vi "FRC ADIS16460 Example.vi"() -> ()   [LabVIEW 2015]
doc: "SimpleGyro Example\n\nThis example shows how to use a SimpleGyro sensor connected to the SPI port on the RoboRIO.\n\nThis example expects a USB cable connected from your development PC to the Type B USB Jack (next to the power input) on the roboRIO."
uses:
  <vilib>/Rock Robotics/SystemInterfaces/spilib/spi_bus.ctl
  ADI MXP IMU/FRC ADIS16460.lvlib
panel:
  out "IMU Data":T1
  out "IMU AHRS":cluster{"Pitch":dbl, "Roll":dbl}
  out "Sensor Ready?":bool
  out "IMU Angle Delta":cluster{"X":dbl, "Y":dbl, "Z":dbl}
  in  "Reset Angle?":bool
  out "Device Found?":bool
  in  "stop":bool
  # "FRC Analog Devices ADIS16460 IMU Example"
  # "FRC ADI MXP Placement"
  # "Raw IMU Output Data"
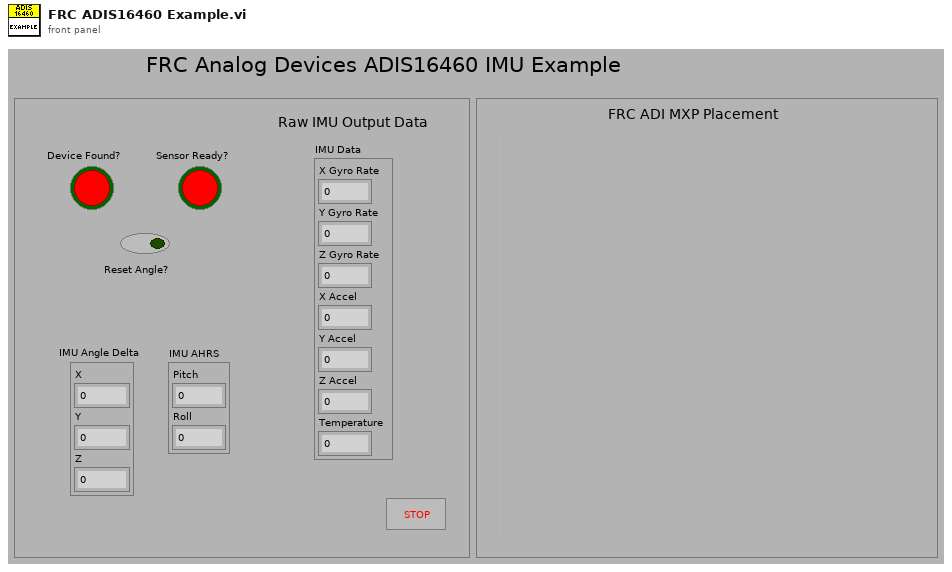
[diagram p1: front panel]
types:
  T1 = cluster{"X Gyro Rate":dbl, "Y Gyro Rate":dbl, "Z Gyro Rate":dbl, "X Accel":dbl, "Y Accel":dbl, "Z Accel":dbl, "Temperature":dbl}
  T2 = typedef "spi_bus.ctl" = enum16{"SPI On-Board, CS0", "SPI On-Board, CS1", "SPI On-Board, CS2", "SPI On-Board, CS3", "SPI MXP", "Invalid"}
  T3 = typedef "FRC ADIS16460.lvlib/WPI_ADIS16460_InterruptDevRef.ctl" = cluster{"ADI IMU DevRef":T4, "InterruptRef":T5}
  T4 = typedef "FRC ADIS16460.lvlib/WPI_ADIS16460_DevRef.ctl" = cluster{"DevStatus":errorcluster, "Handle":i32, "SPI Bus":T2, "Device Found":bool, "Device Ready":bool, "Yaw Axis":enum16{"X", "Y", "Z"}, "AHRS Algorithm":enum16{"Complementary", "Madgwick"}}
  T5 = typedef "WPI_InterruptRef.ctl" = cluster{"DevStatus":errorcluster, "InterruptIndex":T6}
  T6 = typedef "FPGA_InterruptIndex.ctl" = enum8{"0", "1", "2", "3", "4", "5", "6", "7", "Invalid"}
  T7 = cluster{"X Angle":dbl, "Y Angle":dbl, "Z Angle":dbl}
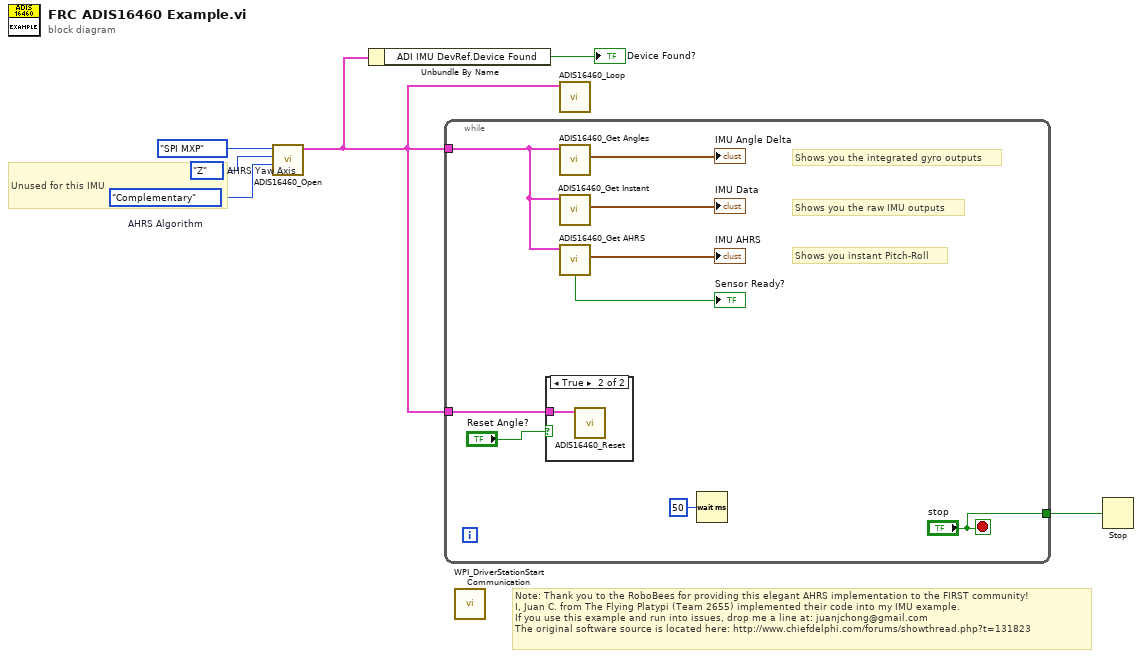
[diagram p0: block diagram]
diagram:
  w1 = enum16{"Complementary", "Madgwick"}."Complementary"  # AHRS Algorithm
  w2 = enum16{"X", "Y", "Z"}."Z"  # AHRS Yaw Axis
  # "Unused for this IMU"
  # "Note: Thank you to the RoboBees for providing this elegant AHRS implementation to the FIRST community!\nI, Juan C. from The Flying Platypi (Team 2655) implemented their code into my IMU example.\nIf you use this example and run into issues, drop me a line at: juanjchong@gmail.com\nThe original software source is located here: http://www.chiefdelphi.com/forums/showthread.php?t=131823"
  n1 = call "ADIS16460_Open.vi"("AHRS Algorithm"=w1, "Yaw Axis"=w2, "SPI Chip Select"=spi_bus."SPI MXP") -> ("ADI IMU Interrupt DevRef"=w3:T3)  [unwired: 7 in, 1 out]
  n2 = Unbundle By Name(w3) -> ("ADI IMU DevRef.Device Found"=→"Device Found?":bool)
  n3 = while {
    tunnel: w3 -> [w7]
    tunnel: ["stop"] -> w5
    tunnel: w3 -> [w14]
    stop <- "stop" stop-if-true
    # "Shows you the integrated gyro outputs"
    # "Shows you the raw IMU outputs"
    # "Shows you instant Pitch-Roll"
    n4 = case shown="True" "Reset Angle?" {
      tunnel: w14 -> [_ w16]
      frame False {
      }
      frame True {
        n5 = call "ADIS16460_Reset.vi"("ADI IMU Interrupt DevRef"=w16) -> ()  [unwired: 9 in, 2 out]
      }
    }
    n6 = call "ADIS16460_Get Angles.vi"("ADI IMU Interrupt DevRef"=w7) -> ("IMU Angles"=→"IMU Angle Delta":T7)  [unwired: 7 in, 3 out]
    n7 = call "ADIS16460_Get Instant.vi"("ADI IMU Interrupt DevRef"=w7) -> ("IMU Data"=→"IMU Data":T1)  [unwired: 7 in, 3 out]
    n8 = call "ADIS16460_Get AHRS.vi"("ADI IMU Interrupt DevRef"=w7) -> ("IMU AHRS OUT"=→"IMU AHRS":cluster{"Pitch":dbl, "Roll":dbl}, "Sensor Ready Out"=→"Sensor Ready?":bool)  [unwired: 7 in, 2 out]
    n9 = Wait (ms)(milliseconds to wait=u32 50) -> ()  [unwired: 1 out]
  }
  n10 = call <vilib>:"WPI_DriverStationStart Communication.vi"() -> ()  [unwired: 12 in]
  n11 = call "ADIS16460_Loop.vi"("ADI IMU Interrupt DevRef"=w3) -> ()  [unwired: 9 in, 2 out]
  n12 = Stop(stop? (T)=w5) -> ()
